vi "HFRR ADV v044.vi"() -> ()   [LabVIEW 2025] (continued)
          frame #3 {
          }
          frame #4 {
          }
          frame #5 {
          }
          frame #6 {
            # "CAL;END"
          }
          frame #7 {
            w857 = 0.0 ("x")
            w858 = 60.0 ("x")
            n824 = local read "Temperature diff"() -> (w861:dbl)
            n825 = local read "Air 60deg temp"() -> (w860:dbl)
            n826 = local read "Air 0deg temp"() -> (w859:dbl)
            n827 = Add(x=w858, y=w861) -> (x+y=w868:dbl)
            n828 = Subtract(x=w858, y=w861) -> (x-y=w867:dbl)
            n829 = Add(x=w857, y=w861) -> (x+y=w866:dbl)
            n830 = Subtract(x=w857, y=w861) -> (x-y=w865:dbl)
            n831 = In Range and Coerce(upper limit=w868, x=w860, lower limit=w867) -> (In Range?=w864:bool)  [unwired: 1 out]
            n832 = In Range and Coerce(upper limit=w866, x=w859, lower limit=w865) -> (In Range?=w863:bool)  [unwired: 1 out]
            n833 = And(x=w864, y=w863) -> (x .and. y?=w862:bool)
            n834 = case shown="True" w862 {
              frame False {
                n835 = property on="Accept & Save Air Temperature step 4" class="Bool (strict)"("DisabledEnum"=T19."Disabled" ("Disabled")) -> ()  [unwired: 2 in, 2 out]
                n836 = local write "Air Temperature Calibration"(enum32{"True", "Fail"}."Fail" ("Sample Temperature Calibration  2")) -> ()
              }
              frame True {
                n837 = local write "Air Temperature Calibration"(enum32{"True", "Fail"}."True" ("Sample Temperature Calibration  2")) -> ()
                n838 = property on="Accept & Save Air Temperature step 4" class="Bool (strict)"("DisabledEnum"=T19."Enabled" ("Disabled")) -> ()  [unwired: 2 in, 2 out]
              }
            }
          }
          frame #8 {
            # "CAL;END"
          }
          frame #9 {
            n839 = local write "Tab Control 4"(T14."Air Step 4" ("Tab Control 4")) -> ()
          }
        }
      }
      event "Back Stroke step main temperature": Value Change {
        n840 = event-data() -> ()  [unwired: 1 in, 6 out]
        n841 = stacked-sequence {
          frame #0 {
            n842 = Wait (ms)(milliseconds to wait=u32 1000) -> ()  [unwired: 1 out]
          }
          frame #1 {
            # "CAL;END"
            n843 = local write "Due Write"("CAL;END" ("Command")) -> ()
          }
          frame #2 {
            n844 = Wait (ms)(milliseconds to wait=u32 1000) -> ()  [unwired: 1 out]
          }
          frame #3 {
            # "CAL;END"
            n845 = local write "Due Write"("CAL;END" ("Command")) -> ()
          }
          frame #4 {
            n846 = local write "Temperature Selection"(T15."Default" ("Temperature Selection")) -> ()
            n847 = local write "Calibration Selection"(T10."Default" ("Calibration Selection")) -> ()
            n848 = local write "Main Calibration Tab"(T9."Main" ("Main Calibration Tab")) -> ()
            n849 = local write "Tab Control 4"(T14."Main" ("Tab Control 4")) -> ()
          }
        }
      }
      event "TEMPERATURE STEP  Back 4", "TEMPERATURE STEP 1 Back 3", "TEMPERATURE STEP  Back 3", "TEMPERATURE STEP 1 Back 2", "Back Air TEMPERATURE Step 4", "Back SAMPLE TEMPERATURE Step 4": Value Change {
        # "Back Stroke step main temperature"
        n850 = event-data() -> ()  [unwired: 1 in, 6 out]
        n851 = stacked-sequence {
          frame #0 {
            n852 = Wait (ms)(milliseconds to wait=u32 1000) -> ()  [unwired: 1 out]
          }
          frame #1 {
            # "CAL;END"
            n853 = local write "Due Write"("CAL;END" ("Command")) -> ()
          }
          frame #2 {
            n854 = Wait (ms)(milliseconds to wait=u32 1000) -> ()  [unwired: 1 out]
          }
          frame #3 {
            # "CAL;END"
            n855 = local write "Due Write"("CAL;END" ("Command")) -> ()
          }
          frame #4 {
            # "TEMPERATURE STEP  Back 4"
            n856 = local write "Main Calibration Tab"(T9."Temperature" ("Main Calibration Tab")) -> ()
            n857 = local write "Temperature Selection"(T15."Default" ("Temperature Selection")) -> ()
            n858 = local write "Tab Control 4"(T14."Main" ("Tab Control 4")) -> ()
            n859 = local write "Calibration Selection"(T10."Default" ("Calibration Selection")) -> ()
          }
        }
      }
      event "FF BACK", "FF BACK 2", "FF BACK 3", "FF BACK 4", "FF BACK 5", "FF BACK 6": Value Change {
        n860 = event-data() -> ()  [unwired: 1 in, 6 out]
        n861 = stacked-sequence {
          frame #0 {
            n862 = Wait (ms)(milliseconds to wait=u32 1000) -> ()  [unwired: 1 out]
          }
          frame #1 {
            n863 = local write "Due Write"("VC;0") -> ()
          }
          frame #2 {
            n864 = Wait (ms)(milliseconds to wait=u32 1000) -> ()  [unwired: 1 out]
          }
          frame #3 {
            n865 = local write "Due Write"("VC;0") -> ()
          }
          frame #4 {
            w894 = FALSE
            n866 = local write "FF BACK 2"(w894) -> ()
            n867 = local write "FF BACK 3"(w894) -> ()
            n868 = local write "FF BACK 4"(w894) -> ()
            n869 = local write "FF BACK 5"(w894) -> ()
            n870 = local write "FF BACK 6"(w894) -> ()
            n871 = local write "FF BACK"(w894) -> ()
          }
          frame #5 {
            n872 = local write "Temperature Selection"(T15."Default" ("Temperature Selection")) -> ()
            n873 = local write "Calibration Selection"(T10."Default" ("Calibration Selection")) -> ()
            n874 = local write "Friction Force Tab"(T13."Page 1" ("Friction Force Tab")) -> ()
            n875 = local write "Main Calibration Tab"(T9."Main" ("Main Calibration Tab")) -> ()
            n876 = property on="Tab Control 6" class="TabCtl (strict)"("Visible"=FALSE) -> ()  [unwired: 2 in, 2 out]
            n877 = property on="Friction Force Calibration Result Tab" class="TabCtl (strict)"("Visible"=FALSE) -> ()  [unwired: 2 in, 2 out]
          }
        }
      }
      event "Accept & Save FF": Value Change {
        n878 = event-data() -> ()  [unwired: 1 in, 6 out]
        n879 = stacked-sequence {
          frame #0 {
            n880 = Wait (ms)(milliseconds to wait=u32 1000) -> ()  [unwired: 1 out]
          }
          frame #1 {
            n881 = local write "Due Write"("VC;0") -> ()
          }
          frame #2 {
            n882 = Wait (ms)(milliseconds to wait=u32 1000) -> ()  [unwired: 1 out]
          }
          frame #3 {
            n883 = local write "Due Write"("VC;0") -> ()
          }
          frame #4 {
            w905 = FALSE
            n884 = local write "FF BACK 2"(w905) -> ()
            n885 = local write "FF BACK 3"(w905) -> ()
            n886 = local write "FF BACK 4"(w905) -> ()
            n887 = local write "FF BACK 5"(w905) -> ()
            n888 = local write "FF BACK 6"(w905) -> ()
            n889 = local write "FF BACK"(w905) -> ()
          }
          frame #5 {
            n890 = Get Date/Time In Seconds() -> (seconds since 1Jan1904=w908:timestamp)
            n891 = Format Into String(format string="%<%I:%M:%S:%p %d:%B:%Y>T", w908) -> (resulting string=w906:string)  [unwired: 2 in, 1 out]
            n892 = local write "FRICTION CALIBRATION"(w906) -> ()
          }
          frame #6 {
            n893 = local write "Temperature Selection"(T15."Default" ("Temperature Selection")) -> ()
            n894 = local write "Calibration Selection"(T10."Default" ("Calibration Selection")) -> ()
            n895 = local write "Friction Force Tab"(T13."Page 1" ("Friction Force Tab")) -> ()
            n896 = local write "Main Calibration Tab"(T9."Main" ("Main Calibration Tab")) -> ()
            n897 = local write "Save Button"(TRUE ("Save Button")) -> ()
            n898 = property on="Tab Control 6" class="TabCtl (strict)"("Visible"=FALSE) -> ()  [unwired: 2 in, 2 out]
            n899 = property on="Friction Force Calibration Result Tab" class="TabCtl (strict)"("Visible"=FALSE) -> ()  [unwired: 2 in, 2 out]
          }
        }
      }
      event "FF CONTINUE": Value Change {
        n900 = event-data() -> ()  [unwired: 1 in, 6 out]
        n901 = local write "FF CONTINUE"(FALSE ("FF CONTINUE")) -> ()
        n902 = local write "Friction Force Tab"(T13."Page 2" ("Friction Force Tab")) -> ()
      }
      event "FF CONTINUE 2": Value Change {
        n903 = event-data() -> ()  [unwired: 1 in, 6 out]
        n904 = local write "FF CONTINUE 2"(FALSE ("FF CONTINUE")) -> ()
        n905 = local write "Friction Force Tab"(T13."Page 3" ("Friction Force Tab")) -> ()
      }
      event "FF CONTINUE 3": Value Change {
        n906 = event-data() -> ()  [unwired: 1 in, 6 out]
        n907 = local write "FF CONTINUE 3"(FALSE ("FF CONTINUE")) -> ()
        n908 = local write "Friction Force Tab"(T13."Page 4" ("Friction Force Tab")) -> ()
      }
      event "FF CONTINUE 4": Value Change {
        n909 = event-data() -> ()  [unwired: 1 in, 6 out]
        n910 = local write "FF CONTINUE 4"(FALSE ("FF CONTINUE")) -> ()
        n911 = local write "Friction Force Tab"(T13."Page 5" ("Friction Force Tab")) -> ()
        n912 = property on="Friction Force Calibration Result Tab" class="TabCtl (strict)"("Visible"=FALSE) -> ()  [unwired: 2 in, 2 out]
      }
      event "FF CONTINUE 5": Value Change {
        n913 = event-data() -> ()  [unwired: 1 in, 6 out]
        n914 = local write "FF CONTINUE 5"(FALSE ("FF CONTINUE")) -> ()
        n915 = local write "Friction Force Tab"(T13."Page 6" ("Friction Force Tab")) -> ()
        n916 = property on="Friction Force Calibration Result Tab" class="TabCtl (strict)"("Visible"=FALSE) -> ()  [unwired: 2 in, 2 out]
        n917 = property on="Tab Control 6" class="TabCtl (strict)"("Visible"=FALSE) -> ()  [unwired: 2 in, 2 out]
      }
      event "Stroke Report Button": Value Change {
        n918 = event-data() -> ()  [unwired: 1 in, 6 out]
        n919 = local read "Point 5 - 1.0 mm"() -> (w930:bool)
        n920 = case shown="False" w930 {
          tunnel: [0.8 1.0] -> w929
          frame False {
          }
          frame True {
          }
        }
        n921 = local read "Machine Serial Number"() -> (w933:string)
        n922 = local read "USERNAME"() -> (w931:string)
        n923 = local write "Stroke Report Button"(FALSE ("Stroke Report Button")) -> ()
        n924 = call "Stroke Calibration Report.vi"("measured_value"=w929, "operator_name"=w931, "Instrument_serial Number"=w933) -> ()  [unwired: 7 in, 2 out]
      }
      event "Sample Report Button": Value Change {
        n925 = event-data() -> ()  [unwired: 1 in, 6 out]
        n926 = local read "Machine Serial Number"() -> (w939:string)
        n927 = local read "Sample 0deg temp"() -> (w936:dbl)
        n928 = local read "Sample 60deg temp"() -> (w937:dbl)
        n929 = local read "USERNAME"() -> (w938:string)
        n930 = call "Temperature Calibration Report.vi"("measured_60"=w937, "measured_zero"=w936, "operator_name"=w938, "Instrument_serial Number"=w939) -> ()  [unwired: 6 in, 2 out]
        n931 = local write "Sample Report Button"(FALSE ("Sample Report Button")) -> ()
      }
      event "Report Button FF": Value Change {
        n932 = event-data() -> ()  [unwired: 1 in, 6 out]
        n933 = local read "FF PASS"() -> (w944:bool)
        n934 = local read "Machine Serial Number"() -> (w947:string)
        n935 = Select(t="PASS", s=w944, f="FAIL") -> (s? t:f=w941:string)
        n936 = local read "USERNAME"() -> (w946:string)
        n937 = call "FF Calibration Report.vi"("pass_or_fail"=w941, "operator_name"=w946, "Instrument_serial Number"=w947) -> ()  [unwired: 7 in, 2 out]
        n938 = local write "Report Button FF"(FALSE ("Sample Report Button")) -> ()
      }
      event "Air Temperature Report Button": Value Change {
        n939 = event-data() -> ()  [unwired: 1 in, 6 out]
        n940 = local read "Machine Serial Number"() -> (w952:string)
        n941 = local read "Air 0deg temp"() -> (w949:dbl)
        n942 = local read "Air 60deg temp"() -> (w950:dbl)
        n943 = local read "USERNAME"() -> (w951:string)
        n944 = call "Air Temperature Calibration Report.vi"("measured_60"=w950, "measured_zero"=w949, "operator_name"=w951, "Instrument_serial Number"=w952) -> ()  [unwired: 6 in, 2 out]
        n945 = local write "Air Temperature Report Button"(FALSE ("Sample Report Button")) -> ()
      }
      event "Quit": Value Change {
        n946 = event-data() -> ()  [unwired: 1 in, 6 out]
      }
    }
    n947 = Wait (ms)(milliseconds to wait=u32 100) -> ()  [unwired: 1 out]
  }
  n948 = while {
    shift-right: [w955] -> _
    shift-left: "Enum - Selector" -> [w956]
    stop <- w957 stop-if-true
    # "Auto Start Logic Loop"
    n949 = case shown="\"Maintain Stage\"" w956 {
      tunnel: [w960 w966 w994 w1029 w1059 Auto_Start_enum."Exit" ("Enum - Selector") Auto_Start_enum."Init" ("Enum - Selector")] -> w955
      frame "Init", Default {
        n950 = local read "Auto Start Test"() -> (w959:bool)
        n951 = Select(t=Auto_Start_enum."Humidity & Temperature On" ("Enum - Selector"), s=w959, f=Auto_Start_enum."Init") -> (s? t:f=w960:T17)
      }
      frame "Humidity & Temperature On" {
        n952 = stacked-sequence {
          tunnel: [_ _ _ _ _ _ Auto_Start_enum."Reach point" ("Enum - Selector")] -> w963
          frame #0 {
            w968 = T19."Disabled and Grayed Out" ("Disabled")
            w969 = TRUE ("Heater Button")
            n953 = property on="Humidity" class="Bool (strict)"("DisabledEnum"=w968) -> ()  [unwired: 2 in, 2 out]
            n954 = property on="Heater Button" class="Bool (strict)"("DisabledEnum"=w968) -> ()  [unwired: 2 in, 2 out]
            n955 = local write "Heater Button"(w969) -> ()
            n956 = local write "Humidity"(w969) -> ()
            n957 = property on="Heater Button" class="Bool (strict)"("Val(Sgnl)"=TRUE ("Value (Signaling)")) -> ()  [unwired: 2 in, 2 out]
          }
          frame #1 {
            n958 = Wait (ms)(milliseconds to wait=u32 3000) -> ()  [unwired: 1 out]
          }
          frame #2 {
            n959 = local read "Set Temp"() -> (w975:dbl)
            n960 = Number To Fractional String(number=w975, precision (6)=i16 2) -> (F-format string=w972:string)  [unwired: 2 in]
            n961 = Concatenate Strings("ST;" ("Command"), w972) -> (w973:string)
            n962 = local write "Due Write"(w973) -> ()
          }
          frame #3 {
            n963 = Wait (ms)(milliseconds to wait=u32 1500) -> ()  [unwired: 1 out]
          }
          frame #4 {
            (unwired) i16 2 ("precision (6)")
            n964 = local read "WriteHumidity"() -> (w977:string[])
            n965 = local read "Set Rh"() -> (w980:dbl)
            n966 = Number To Fractional String(number=w980) -> (F-format string=w981:string)  [unwired: 3 in]
            n967 = Concatenate Strings("M;" ("new element/subarray"), w981) -> (w982:string)
            n968 = Insert Into Array(array=w977, new element=w982) -> (w978:string[])  [unwired: 1 in]
            n969 = local write "WriteHumidity"(w978) -> ()
            n970 = local write "Due Write"("HE;1" ("Command")) -> ()
          }
          frame #5 {
            n971 = Wait (ms)(milliseconds to wait=u32 1500) -> ()  [unwired: 1 out]
          }
          frame #6 {
            w985 = TRUE ("Reach point temp")
            n972 = local write "Reach point Humidity"(w985) -> ()
            n973 = local write "Reach point temp"(w985) -> ()
          }
        }
        n974 = local read "Auto Start Test"() -> (w965:bool)
        n975 = Not(x=w965) -> (.not. x?=w964:bool)
        n976 = Select(t=Auto_Start_enum."close", s=w964, f=w963) -> (s? t:f=w966:T17)
      }
      frame "Reach point" {
        w995 = TRUE ("PAUSE")
        w1003 = 1.0 ("y")
        w1006 = 1.0 ("y")
        n977 = local read "Set Temp"() -> (w988:dbl)
        n978 = local read "Set Humidity:"() -> (w1002:dbl)
        n979 = local read "Humidity ( %RH )"() -> (w1007:dbl)
        n980 = Add(x=w988, y=w1006) -> (x+y=w1005:dbl)
        n981 = Subtract(x=w988, y=w1006) -> (x-y=w1004:dbl)
        n982 = Add(x=w1002, y=w1003) -> (x+y=w1001:dbl)
        n983 = Subtract(x=w1002, y=w1003) -> (x-y=w1000:dbl)
        n984 = local read "TEMP"() -> (w1008:dbl)
        n985 = In Range and Coerce(upper limit=w1001, x=w1007, lower limit=w1000) -> (In Range?=w989:bool)  [unwired: 1 out]
        n986 = In Range and Coerce(upper limit=w1005, x=w1008, lower limit=w1004) -> (In Range?=w990:bool)  [unwired: 1 out]
        n987 = disable-structure shown="Enabled" {
          disable-tunnel: w989 -> [w1009 _]
          disable-tunnel: [w1009 TRUE] -> w987
          frame Disabled {
            n988 = case shown="True" w1009 {
              frame False {
              }
              frame True {
                n989 = case shown="True" "Reach point Humidity" {
                  selector: "Reach point Humidity" -> [_ w1015]
                  frame False {
                  }
                  frame True {
                    n990 = local read "EVENT LOG"() -> (w1012:string)
                    n991 = Not(x=w1015) -> (.not. x?=w1014:bool)
                    n992 = local write "Reach point Humidity"(w1014) -> ()
                    n993 = call "Event Log.vi"("Content"="Target Humidity reached", "EVENT LOG"=w1012) -> ("EVENT LOG"=w1013:string)  [unwired: 8 in, 1 out]
                    n994 = local write "EVENT LOG"(w1013) -> ()
                  }
                }
              }
            }
          }
          frame Enabled {
          }
        }
        n995 = case shown="True" w990 {
          frame False {
          }
          frame True {
            n996 = case shown="True" "Reach point temp" {
              selector: "Reach point temp" -> [_ w1022]
              frame False {
              }
              frame True {
                n997 = local read "EVENT LOG"() -> (w1019:string)
                n998 = Not(x=w1022) -> (.not. x?=w1021:bool)
                n999 = local write "Reach point temp"(w1021) -> ()
                n1000 = call "Event Log.vi"("Content"="Target Temperature reached", "EVENT LOG"=w1019) -> ("EVENT LOG"=w1020:string)  [unwired: 8 in, 1 out]
                n1001 = local write "EVENT LOG"(w1020) -> ()
              }
            }
          }
        }
        n1002 = local read "Auto Start Test"() -> (w993:bool)
        n1003 = And(x=w990, y=w987) -> (x .and. y?=w999:bool)
        n1004 = Select(t=Auto_Start_enum."Maintain Stage" ("Enum - Selector"), s=w999, f=Auto_Start_enum."Reach point" ("Enum - Selector")) -> (s? t:f=w996:T17)
        n1005 = Not(x=w993) -> (.not. x?=w992:bool)
        n1006 = Select(t=Auto_Start_enum."close", s=w992, f=w996) -> (s? t:f=w994:T17)
        n1007 = call "ELAPSED TIMER VI.vi"("RESET"=w995, "PAUSE"=w995) -> ()  [unwired: 7 in, 3 out]
      }
      frame "Maintain Stage" {
        w1037 = 2.0 ("y")
        w1036 = 1.0 ("y")
        # "Humidity and temperature set point has stabilized."
        # "Humidity and  temperatures Set Point  have been reached"
        n1008 = local read "Set Temp"() -> (w1024:dbl)
        n1009 = local read "Set Humidity:"() -> (w1040:dbl)
        n1010 = local read "Humidity ( %RH )"() -> (w1043:dbl)
        n1011 = Add(x=w1024, y=w1036) -> (x+y=w1042:dbl)
        n1012 = Subtract(x=w1024, y=w1036) -> (x-y=w1041:dbl)
        n1013 = local read "TEMP"() -> (w1044:dbl)
        n1014 = Add(x=w1040, y=w1037) -> (x+y=w1039:dbl)
        n1015 = Subtract(x=w1040, y=w1037) -> (x-y=w1038:dbl)
        n1016 = In Range and Coerce(upper limit=w1042, x=w1044, lower limit=w1041) -> (In Range?=w1035:bool)  [unwired: 1 out]
        n1017 = In Range and Coerce(upper limit=w1039, x=w1043, lower limit=w1038) -> ()  [unwired: 2 out]
        n1018 = And(x=w1035, y=TRUE) -> (x .and. y?=w1034:bool)
        n1019 = Not(x=w1034) -> (.not. x?=w1033:bool)
        n1020 = call "ELAPSED TIMER VI.vi"("TARGET"=60.0, "RESET"=w1033, "PAUSE"=FALSE) -> ("ELAPSED INDICATION"=w1030:bool)  [unwired: 6 in, 2 out]
        n1021 = case shown="True" w1030 {
          tunnel: w1030 -> [_ w1047]
          tunnel: [Auto_Start_enum."Maintain Stage" ("Enum - Selector") w1046] -> w1028
          frame False {
          }
          frame True {
            n1022 = stacked-sequence {
              tunnel: w1047 -> [_ _ _ _ _]
              tunnel: [_ _ _ _ Auto_Start_enum."Start Stage" ("Enum - Selector")] -> w1046
              frame #0 {
                n1023 = local read "EVENT LOG"() -> (w1049:string)
                n1024 = call "Event Log.vi"("Content"="Temperature set point has stabilized.", "EVENT LOG"=w1049) -> ("EVENT LOG"=w1050:string)  [unwired: 8 in, 1 out]
                n1025 = local write "EVENT LOG"(w1050) -> ()
              }
              frame #1 {
                n1026 = Wait (ms)(milliseconds to wait=u32 100) -> ()  [unwired: 1 out]
              }
              frame #2 {
                n1027 = local read "EVENT LOG"() -> (w1054:string)
                n1028 = call "Event Log.vi"("Content"="Auto Test Started", "EVENT LOG"=w1054) -> ("EVENT LOG"=w1055:string)  [unwired: 8 in, 1 out]
                n1029 = local write "EVENT LOG"(w1055) -> ()
                n1030 = local write "FRICVALZ 4"(TRUE ("FRICVALZ 4")) -> ()
              }
              frame #3 {
                w1056 = TRUE ("RUN")
                n1031 = local write "RUN"(w1056) -> ()
                n1032 = property on="Auto Start Temp" class="Bool (strict)"("Val(Sgnl)"=w1056) -> ()  [unwired: 2 in, 2 out]
                "Auto Start Temp" <- w1056
              }
              frame #4 {
              }
            }
          }
        }
        n1033 = local read "Auto Start Test"() -> (w1027:bool)
        n1034 = Not(x=w1027) -> (.not. x?=w1026:bool)
        n1035 = Select(t=Auto_Start_enum."close", s=w1026, f=w1028) -> (s? t:f=w1029:T17)
      }
      frame "Start Stage" {
        w1058 = TRUE ("PAUSE")
        n1036 = local read "Auto Start Test"() -> (w1063:bool)
        n1037 = Not(x=w1063) -> (.not. x?=w1062:bool)
        n1038 = Select(t=Auto_Start_enum."close" ("Enum - Selector"), s=w1062, f=Auto_Start_enum."Start Stage" ("Enum - Selector")) -> (s? t:f=w1059:T17)
        n1039 = call "ELAPSED TIMER VI.vi"("RESET"=w1058, "PAUSE"=w1058) -> ()  [unwired: 7 in, 3 out]
      }
      frame "close" {
        w1066 = FALSE ("Heater Button")
        n1040 = local write "RUN"(w1066) -> ()
        n1041 = local write "Heater Button"(w1066) -> ()
        n1042 = local write "Humidity"(w1066) -> ()
        n1043 = local write "Auto Start Test"(w1066) -> ()
        n1044 = property on="Heater Button" class="Bool (strict)"("Val(Sgnl)"=FALSE ("Value (Signaling)")) -> ()  [unwired: 2 in, 2 out]
        n1045 = local write "Humidity 2"(TRUE ("Humidity")) -> ()
      }
      frame "Exit" {
      }
    }
    n1046 = Wait (ms)(milliseconds to wait=u32 100) -> ()  [unwired: 1 out]
    n1047 = local read "Quit"() -> (w957:bool)
  }
  n1048 = property on="Service Password Log" class="Str"("Visible"=w26) -> ()  [unwired: 2 in, 2 out]
  n1049 = property on="Password 3" class="Clust (strict)"("Visible"=w26) -> ()  [unwired: 2 in, 2 out]
  n1050 = while {
    stop <- w1095 stop-if-true
    w1078 = errorcluster {"status"=FALSE, "code"=0, "source"=""} ("error in (no error) 3")
    # "this loop is for manual report generation"
    n1051 = local read "Confirm Measrurement"() -> (w1077:bool)
    n1052 = case shown="True" w1077 {
      selector: w1077 -> [_ w1185]
      tunnel: errorcluster {"status"=FALSE, "code"=0, "source"=""} ("error in (no error) 3") -> [_ w1186]
      tunnel: [_ w1184] -> _
      frame False {
      }
      frame True {
        n1053 = stacked-sequence {
          tunnel: w1186 -> [_ w1219 _]
          tunnel: w1185 -> [_ _ w1326]
          tunnel: [_ w1207 _] -> w1184
          frame #0 {
            n1054 = String To Path(string="C:\\LAB-IQ\\Image Calibrate v01.dcf") -> (path=w1189:path)
            n1055 = Open/Create/Replace File ("Open File")(file path (use dialog)=w1189) -> (refnum out=w1190:refnum<file>)  [unwired: 5 in, 2 out]
            n1056 = for {
              N: 4 -> [_]
              tunnel: w1190 -> [w1196]
              i -> [w1192]
              n1057 = Read from Text File ("Read File")(file (use dialog)=w1196) -> (text=w1197:string)  [unwired: 3 in, 3 out]
              n1058 = String Subset(string=w1197, offset (0)=6, length (rest)=10 ("length (rest)")) -> (substring=w1193:string)
              n1059 = Fract/Exp String To Number(string=w1193) -> (number=w1191:dbl)  [unwired: 3 in, 1 out]
              n1060 = case shown="3" w1192 {
                tunnel: w1191 -> [w1198 w1199 _ w1200 _]
                frame 0 {
                  n1061 = local write "5x Gain"(w1198) -> ()
                }
                frame 1 {
                  n1062 = local write "10x Gain"(w1199) -> ()
                }
                frame 2 {
                }
                frame 3 {
                  n1063 = local write "100x gain"(w1200) -> ()
                }
                frame 4, Default {
                }
              }
            }
          }
          frame #1 {
            n1064 = local read "TEST STANDARD"() -> (w1202:T5)
            n1065 = case shown="\"ISO 12156\"" w1202 {
              tunnel: ["ASTM D6079" "ISO 12156"] -> w1201
              frame "ASTM D6079", Default {
              }
              frame "ISO 12156" {
              }
            }
            n1066 = call "IMAGE ANALYSIS.vi"("Enum"=POST_ANALYSIS_ENUM."GET MEASUREMENTS", "error in"=w1219) -> ("error out"=w1226:errorcluster)  [unwired: 8 in, 1 out]
            n1067 = local read "Magnification :"() -> (w1212:string)
            n1068 = call "Stall Data Flow.vim"("value in"=w1226, "milliseconds to wait"=u32 1000) -> ("value out"=w1225:errorcluster)  [unwired: 1 out]
            n1069 = local read "Test File List :"() -> (w1223:string)
            n1070 = case shown="\"10x\"" w1212 {
              tunnel: [w1262 w1263] -> w1210
              frame "5x", Default {
                n1071 = local read "5x Gain"() -> (w1262:dbl)
              }
              frame "10x" {
                # "5x"
                n1072 = local read "10x Gain"() -> (w1263:dbl)
              }
            }
            n1073 = call "IMAGE ANALYSIS.vi"("Enum"=POST_ANALYSIS_ENUM."READ", "error in"=w1225) -> ("error out"=w1222:errorcluster, "data out"=w1213:string)  [unwired: 8 in]
            n1074 = Match Pattern(string=w1213, regular expression="\"type\": ") -> (after substring=w1217:string)  [unwired: 1 in, 3 out]
            n1075 = call "IMAGE PATH CREATION PY.vi"("error in (no error)"=w1222, "File Name :"=w1223) -> ("error out"=w1221:errorcluster, "File Path"=w1209:path, "File Path String:"=w1204:string)  [unwired: 7 in]
            n1076 = Match Pattern(string=w1217, regular expression=",") -> (before substring=w1203:string)  [unwired: 1 in, 3 out]
            n1077 = local read "Calibration Tab"() -> (w1206:enum32{"Measrument", "Calibrate"})
            n1078 = call "Stall Data Flow.vim"("value in"=w1221, "milliseconds to wait"=u32 250) -> ("value out"=w1205:errorcluster)  [unwired: 1 out]
            n1079 = Equal?(x=w1203, y="\"rectangle\"") -> (x = y?=w1214:bool)
            n1080 = case shown="False" w1214 {
              tunnel: w1213 -> [w1268 w1323]
              tunnel: w1210 -> [_ w1314]
              tunnel: cluster{"major":dbl, "minor":dbl, "average":dbl} {"major"=0.0, "minor"=0.0, "average"=0.0} -> [w1266 w1310]
              tunnel: [w1265 w1307] -> w1208
              tunnel: w1203 -> [w1267 _]
              tunnel: w1210 -> [w1264 _]
              frame False {
                n1081 = Equal?(x=w1267, y="\"line\"") -> (x = y?=w1269:bool)
                n1082 = case shown="True" w1269 {
                  tunnel: w1268 -> [_ w1284]
                  tunnel: w1266 -> [w1271 w1283]
                  tunnel: [w1271 w1281] -> w1265
                  tunnel: w1264 -> [_ w1280]
                  frame False {
                  }
                  frame True {
                    w1279 = 0.0 ("Major Axis")
                    n1083 = Match Pattern(string=w1284, regular expression="\"length_px\":") -> (after substring=w1282:string)  [unwired: 1 in, 3 out]
                    n1084 = property on="Major Axis" class="DigNum (strict)"("Caption.Text"="") -> ()  [unwired: 2 in, 2 out]
                    n1085 = property on="Minor Axis" class="DigNum (strict)"("Caption.Text"="") -> ()  [unwired: 2 in, 2 out]
                    n1086 = property on="Average" class="DigNum (strict)"("Caption.Text"="Line") -> ()  [unwired: 2 in, 2 out]
                    n1087 = Fract/Exp String To Number(string=w1282, default (0 dbl)=0.0 ("default (0 DBL)")) -> (number=w1278:dbl)  [unwired: 2 in, 1 out]
                    "Pixel Value" <- w1278
                    n1088 = Multiply(x=w1278, y=w1280) -> (x*y=w1291:dbl)
                    n1089 = Multiply(x=w1291, y=1000.0) -> (x*y=w1274:dbl)
                    n1090 = Divide(x=w1274, y=1000.0) -> (x/y=w1277:dbl)
                    n1091 = local write "Measurment (mm)"(w1277) -> ()
                    n1092 = Bundle By Name(cluster=w1283, "average"=w1274) -> (w1281:cluster{"major":dbl, "minor":dbl, "average":dbl})
                    n1093 = Number To Fractional String(number=w1274, precision (6)=i16 1) -> (F-format string=w1273:string)  [unwired: 2 in]
                    n1094 = local write "Minor Axis"(w1279) -> ()
                    n1095 = local write "Major Axis"(w1279) -> ()
                    n1096 = Fract/Exp String To Number(string=w1273) -> (number=w1272:dbl)  [unwired: 3 in, 1 out]
                    n1097 = local write "Average"(w1272) -> ()
                  }
                }
              }
              frame True {
                w1311 = 1000.0 ("y")
                w1317 = 0.0 ("default (0 DBL)")
                n1098 = Match Pattern(string=w1323, regular expression=" \"width_px\":") -> (after substring=w1321:string)  [unwired: 1 in, 3 out]
                n1099 = Match Pattern(string=w1321, regular expression="\"height_px\":") -> (before substring=w1319:string, after substring=w1318:string)  [unwired: 1 in, 2 out]
                n1100 = Fract/Exp String To Number(string=w1319, default (0 dbl)=w1317) -> (number=w1316:dbl)  [unwired: 2 in, 1 out]
                n1101 = Fract/Exp String To Number(string=w1318, default (0 dbl)=w1317) -> (number=w1315:dbl)  [unwired: 2 in, 1 out]
                n1102 = Multiply(x=w1316, y=w1314) -> (x*y=w1313:dbl)
                n1103 = Multiply(x=w1315, y=w1314) -> (x*y=w1312:dbl)
                n1104 = Multiply(x=w1313, y=w1311) -> (x*y=w1297:dbl)
                n1105 = Multiply(x=w1312, y=w1311) -> (x*y=w1295:dbl)
                n1106 = Add(x=w1297, y=w1295) -> (x+y=w1309:dbl)
                n1107 = property on="Major Axis" class="DigNum (strict)"("Caption.Text"="Major Axis") -> ()  [unwired: 2 in, 2 out]
                n1108 = property on="Minor Axis" class="DigNum (strict)"("Caption.Text"="Minor Axis") -> ()  [unwired: 2 in, 2 out]
                n1109 = property on="Average" class="DigNum (strict)"("Caption.Text"="Average") -> ()  [unwired: 2 in, 2 out]
                n1110 = Divide(x=w1309, y=2.0) -> (x/y=w1293:dbl)
                n1111 = Bundle By Name(cluster=w1310, "major"=w1297, "minor"=w1295, "average"=w1293) -> (w1307:cluster{"major":dbl, "minor":dbl, "average":dbl})
                n1112 = Number To Fractional String(number=w1295, precision (6)=i16 1) -> (F-format string=w1302:string)  [unwired: 2 in]
                n1113 = Number To Fractional String(number=w1293, precision (6)=i16 1) -> (F-format string=w1303:string)  [unwired: 2 in]
                n1114 = Number To Fractional String(number=w1297, precision (6)=i16 1) -> (F-format string=w1301:string)  [unwired: 2 in]
                n1115 = Fract/Exp String To Number(string=w1302) -> (number=w1294:dbl)  [unwired: 3 in, 1 out]
                n1116 = Fract/Exp String To Number(string=w1303) -> (number=w1292:dbl)  [unwired: 3 in, 1 out]
                n1117 = Fract/Exp String To Number(string=w1301) -> (number=w1296:dbl)  [unwired: 3 in, 1 out]
                n1118 = local write "Major Axis"(w1296) -> ()
                n1119 = local write "Average"(w1292) -> ()
                n1120 = local write "Minor Axis"(w1294) -> ()
              }
            }
            n1121 = case shown="\"Measrument\", Default" w1206 {
              tunnel: w1209 -> [w1236 _]
              tunnel: w1208 -> [w1235 _]
              tunnel: [w1232 w1261] -> w1207
              tunnel: w1205 -> [w1234 w1261]
              tunnel: w1204 -> [w1233 _]
              tunnel: w1201 -> [w1231 _]
              frame "Measrument", Default {
                n1122 = stacked-sequence {
                  tunnel: w1236 -> [w1254 _]
                  tunnel: w1235 -> [w1252 _]
                  tunnel: w1234 -> [w1250 _]
                  tunnel: w1233 -> [w1249 _]
                  tunnel: [w1244 _] -> w1232
                  tunnel: w1231 -> [w1237 _]
                  frame #0 {
                    n1123 = call "IMAGE ANALYSIS.vi"("Enum"=POST_ANALYSIS_ENUM."SAVE IMAGE", "error in"=w1250, "IMAGE FILE PATH"=w1249) -> ("error out"=w1248:errorcluster)  [unwired: 7 in, 1 out]
                    n1124 = call "Stall Data Flow.vim"("value in"=w1248, "milliseconds to wait"=u32 1000) -> ("value out"=w1239:errorcluster)  [unwired: 1 out]
                    n1125 = local read "Test File List :"() -> (w1256:string)
                    n1126 = call "IMAGE ANALYSIS.vi"("Enum"=POST_ANALYSIS_ENUM."MINIMIZE UI", "error in"=w1239) -> ("error out"=w1246:errorcluster)  [unwired: 8 in, 1 out]
                    n1127 = Bundle By Name(cluster=T26 {"File Name"="", "Test Method"="", "Operator"="", "Fuel Description"="", "Date and time"=""} ("Main Ref"), "Test Method"=w1237, "File Name"=w1256) -> (w1257:T26)
                    n1128 = call "Stall Data Flow.vim"("value in"=w1246, "milliseconds to wait"=u32 1500) -> ("value out"=w1241:errorcluster)  [unwired: 1 out]
                    n1129 = call "duf file read.vi"("error in (no error)"=w1241, "Main Ref"=w1257) -> ("error out"=w1255:errorcluster, "Main Ref 2"=w1253:T26)  [unwired: 8 in]
                    n1130 = call "DETECTION REPORT for manual.vi"("error in (no error)"=w1255, "return value 3"=w1252, "Image File Path"=w1254, "Main Ref"=w1253) -> ("error out"=w1251:errorcluster)  [unwired: 7 in]
                    n1131 = call <vilib>:"Clear Errors.vi"("error in (no error)"=w1251) -> ("error out"=w1242:errorcluster)  [unwired: 5 in, 1 out]
                    n1132 = call "IMAGE ANALYSIS.vi"("Enum"=POST_ANALYSIS_ENUM."MINIMIZE UI", "error in"=w1242) -> ("error out"=w1244:errorcluster)  [unwired: 8 in, 1 out]
                  }
                  frame #1 {
                    n1133 = local write "Main Tab"(T4."HOME" ("Main Tab")) -> ()
                    n1134 = local write "Main Dashboard Buttons"(T1."Home" ("Main Dashboard Buttons")) -> ()
                  }
                }
              }
              frame "Calibrate" {
              }
            }
          }
          frame #2 {
            n1135 = Not(x=w1326) -> (.not. x?=w1325:bool)
            n1136 = local write "Confirm Measrurement"(w1325) -> ()
            n1137 = local read "Calibration Tab"() -> (w1324:enum32{"Measrument", "Calibrate"})
            n1138 = case shown="\"Measrument\", Default" w1324 {
              frame "Measrument", Default {
                (unwired) T21."HOME" ("Main Tab")
                n1139 = local write "Main Tab"(T4."HOME" ("Main Tab")) -> ()
              }
              frame "Calibrate" {
              }
            }
          }
        }
      }
    }
    n1140 = local read "Humidity"() -> (w1069:bool)
    n1141 = local read "Save Change"() -> (w1074:bool)
    n1142 = local read "Calibrate"() -> (w1075:bool)
    n1143 = local read "Auto Start Test"() -> (w1070:bool)
    n1144 = case shown="True" w1075 {
      selector: w1075 -> [_ w1182]
      frame False {
      }
      frame True {
        n1145 = Not(x=w1182) -> (.not. x?=w1181:bool)
        n1146 = local write "Calibrate"(w1181) -> ()
        n1147 = local write "Calibration Tab"(enum32{"Measrument", "Calibrate"}."Calibrate" ("Calibration Tab")) -> ()
      }
    }
    n1148 = case shown="True" w1074 {
      selector: w1074 -> [_ w1126]
      frame False {
      }
      frame True {
        n1149 = stacked-sequence {
          tunnel: w1126 -> [_ _ _ _ w1180]
          frame #0 {
            n1150 = call "IMAGE ANALYSIS.vi"("Enum"=POST_ANALYSIS_ENUM."HIDE UI") -> ()  [unwired: 9 in, 2 out]
          }
          frame #1 {
            n1151 = local read "100x gain"() -> (w1128:dbl)
            n1152 = local read "10x Gain"() -> (w1129:dbl)
            n1153 = local read "5x Gain"() -> (w1130:dbl)
            n1154 = Number To Fractional String(number=w1129, width (-)=i16 4, precision (6)=i16 7) -> (F-format string=w1151:string)  [unwired: 1 in]
            n1155 = Number To Fractional String(number=0.0, width (-)=i16 4, precision (6)=i16 7) -> (F-format string=w1146:string)  [unwired: 1 in]
            n1156 = Number To Fractional String(number=w1128, width (-)=i16 4, precision (6)=i16 7) -> (F-format string=w1134:string)  [unwired: 1 in]
            n1157 = Number To Fractional String(number=w1130, width (-)=i16 10 ("precision (6)"), precision (6)=i16 7) -> (F-format string=w1160:string)  [unwired: 1 in]
            n1158 = Concatenate Strings("[CH1]" ("string"), w1160, " - 5x Gain" ("string"), "\r") -> (w1150:string)
            n1159 = Concatenate Strings("[CH2]" ("string"), w1151, " - 10x Gain" ("string"), "\r") -> (w1149:string)
            n1160 = Concatenate Strings("[CH3]" ("string"), w1146, " - 20x Gain" ("string"), "\r") -> (w1140:string)
            n1161 = Concatenate Strings("[CH4]" ("string"), w1134, " - 100x Gain" ("string"), "\r") -> (w1133:string)
            n1162 = String To Path(string="C:\\LAB-IQ\\Image Calibrate v01.dcf") -> (path=w1163:path)
            n1163 = Concatenate Strings(w1150, w1149, w1140, w1133) -> (w1148:string)
            n1164 = call <vilib>:"Write Characters To File.vi"("append to file? (new file:F)"=FALSE, "character string"=w1148, "file path (dialog if empty)"=w1163) -> ()  [unwired: 2 in, 1 out]
          }
          frame #2 {
            n1165 = String To Path(string="C:\\LAB-IQ\\Image Calibrate v01.dcf") -> (path=w1166:path)
            n1166 = Open/Create/Replace File ("Open File")(file path (use dialog)=w1166) -> (refnum out=w1167:refnum<file>)  [unwired: 5 in, 2 out]
            n1167 = for {
              N: 4 -> [_]
              tunnel: w1167 -> [w1173]
              i -> [w1169]
              n1168 = Read from Text File ("Read File")(file (use dialog)=w1173) -> (text=w1174:string)  [unwired: 3 in, 3 out]
              n1169 = String Subset(string=w1174, offset (0)=6, length (rest)=10 ("length (rest)")) -> (substring=w1170:string)
              n1170 = Fract/Exp String To Number(string=w1170) -> (number=w1168:dbl)  [unwired: 3 in, 1 out]
              n1171 = case shown="3" w1169 {
                tunnel: w1168 -> [w1175 w1176 _ w1177 _]
                frame 0 {
                  n1172 = local write "5x Gain"(w1175) -> ()
                }
                frame 1 {
                  n1173 = local write "10x Gain"(w1176) -> ()
                }
                frame 2 {
                }
                frame 3 {
                  n1174 = local write "100x gain"(w1177) -> ()
                }
                frame 4, Default {
                }
              }
            }
          }
          frame #3 {
            n1175 = call "IMAGE ANALYSIS.vi"("Enum"=POST_ANALYSIS_ENUM."SHOW UI") -> ()  [unwired: 9 in, 2 out]
          }
          frame #4 {
            n1176 = Not(x=w1180) -> (.not. x?=w1179:bool)
            n1177 = local write "Save Change"(w1179) -> ()
          }
        }
      }
    }
    n1178 = case shown="False" w1070 {
      tunnel: w1069 -> [w1096 _]
      frame False {
        n1179 = case shown="True" w1096 {
          frame False {
          }
          frame True {
            n1180 = local read "Set Humidity:"() -> (w1100:dbl)
            n1181 = local read "Set Humidity:"() -> (w1103:dbl)
            n1182 = local read "Humidity ( %RH )"() -> (w1104:dbl)
            n1183 = Subtract(x=w1100, y=2.0) -> (x-y=w1098:dbl)
            n1184 = Add(x=w1103, y=2.0) -> (x+y=w1099:dbl)
            n1185 = In Range and Coerce(upper limit=w1099, x=w1104, lower limit=w1098) -> (In Range?=w1097:bool)  [unwired: 1 out]
            n1186 = case shown="True" w1097 {
              frame False {
              }
              frame True {
                n1187 = case shown="True" "Manual Humididty Reached" {
                  selector: "Manual Humididty Reached" -> [_ w1107]
                  frame False {
                  }
                  frame True {
                    n1188 = Not(x=w1107) -> (.not. x?=w1106:bool)
                    n1189 = local write "Manual Humididty Reached"(w1106) -> ()
                    n1190 = local read "EVENT LOG"() -> (w1109:string)
                    n1191 = call "Event Log.vi"("Content"="Target Humidity reached", "EVENT LOG"=w1109) -> ("EVENT LOG"=w1108:string)  [unwired: 8 in, 1 out]
                    n1192 = local write "EVENT LOG"(w1108) -> ()
                  }
                }
              }
            }
          }
        }
      }
      frame True {
        n1193 = local write "Manual Humididty Reached"(TRUE ("Manual Humididty Reached")) -> ()
      }
    }
    n1194 = local read "Cap Live Image"() -> (w1090:bool)
    n1195 = local read "SCAR MEASURMENT"() -> (w1093:enum32{"Auto Scar", "Manual Scar"})
    n1196 = Equal?(x=w1093, y=enum32{"Auto Scar", "Manual Scar"}."Manual Scar" ("SCAR MEASURMENT")) -> (x = y?=w1091:bool)
    n1197 = And(x=w1091, y=w1090) -> (x .and. y?=w1089:bool)
    n1198 = Wait (ms)(milliseconds to wait=u32 250) -> ()  [unwired: 1 out]
    n1199 = case shown="True" w1089 {
      selector: w1089 -> [_ w1412]
      frame False {
      }
      frame True {
        n1200 = stacked-sequence {
          tunnel: [_ _ _ w1431 _] -> _
          tunnel: w1412 -> [_ _ _ _ w1438]
          frame #0 {
            w1413 = 0.0
            n1201 = local write "Major Axis"(w1413) -> ()
            n1202 = local write "Minor Axis"(w1413) -> ()
            n1203 = local write "Average"(w1413) -> ()
          }
          frame #1 {
            n1204 = call "CAMERA LIVE FEED FGV.vi"("Enum - Menu"=CAMERA_LIVE_FEED_ENUM."CAMERA MINIMIZE") -> ()  [unwired: 9 in, 2 out]
          }
          frame #2 {
            n1205 = local read "Magnification len live scar"() -> (w1417:string)
            n1206 = case shown="\"10x\", Default" w1417 {
              tunnel: ["_10x" "_5x"] -> w1416
              frame "10x", Default {
              }
              frame "5x" {
              }
            }
            n1207 = local read "FILE 3"() -> (w1423:string)
            n1208 = call <vilib>:"Trim Whitespace.vi"("string"="C:\\LAB-IQ\\images\\") -> ("trimmed string"=w1425:string)  [unwired: 1 in]
            n1209 = String To Path(string=w1425) -> (path=w1424:path)
            n1210 = Concatenate Strings(w1423, w1416, ".png" ("string")) -> (w1422:string)
            n1211 = Build Path(base path=w1424, name or relative path=w1422) -> (appended path=w1421:path)
            n1212 = Path To String(path=w1421) -> (string=w1420:string)
            n1213 = call "CAMERA LIVE FEED FGV.vi"("Enum - Menu"=CAMERA_LIVE_FEED_ENUM."CAMERA SAVE", "Image Path"=w1420) -> ("error out"=w1418:errorcluster)  [unwired: 8 in, 1 out]
            n1214 = case shown="No Error" w1418 {
              frame No Error {
                n1215 = One Button Dialog(message="Image saved successfully") -> ()  [unwired: 1 in, 1 out]
              }
              frame Error {
              }
            }
          }
          frame #3 {
            n1216 = call "LIST FILE NAMES.vi"() -> ("error out"=w1433:errorcluster, "filenames"=w1430:string[])  [unwired: 10 in]
            n1217 = call "IMAGE ANALYSIS.vi"("Enum"=POST_ANALYSIS_ENUM."SHOW UI", "error in"=w1433) -> ("error out"=w1431:errorcluster)  [unwired: 8 in, 1 out]
            n1218 = property on="Test File List :" class="CmbBox"("Strings[]"=w1430) -> ()  [unwired: 2 in, 2 out]
          }
          frame #4 {
            (unwired) T25."Report" ("Main Dashboard Buttons")
            (unwired) T27."Report" ("Main Dashboard Buttons")
            n1219 = Not(x=w1438) -> (.not. x?=w1437:bool)
            n1220 = local write "Zoom Factore"(0.0 ("Zoom Factore")) -> ()
            n1221 = local write "Cap Live Image"(w1437) -> ()
            n1222 = local write "Main Tab"(T4."Adv Scar Report" ("Main Tab")) -> ()
            n1223 = property on="Cap Live Image" class="Bool (strict)"("BoolText.Text"="Capture Image" ("Boolean Text.Text")) -> ()  [unwired: 2 in, 2 out]
            n1224 = local write "Main Dashboard Buttons"(T1."Report" ("Main Dashboard Buttons")) -> ()
          }
        }
      }
    }
    n1225 = local read "change Gain"() -> (w1073:bool)
    n1226 = local read "Back Square"() -> (w1072:bool)
    n1227 = case shown="True" w1073 {
      selector: w1073 -> [_ w1117]
      frame False {
      }
      frame True {
        n1228 = stacked-sequence {
          tunnel: w1117 -> [_ w1125]
          frame #0 {
            n1229 = local read "Actual (µm)"() -> (w1121:dbl)
            n1230 = local read "Pixel Value"() -> (w1120:dbl)
            n1231 = local read "Magnification :"() -> (w1119:string)
            n1232 = Divide(x=w1121, y=w1120) -> (x/y=w1118:dbl)
            n1233 = case shown="\"10x\"" w1119 {
              tunnel: w1118 -> [w1122 w1123]
              frame "10x" {
                n1234 = local write "10x Gain"(w1122) -> ()
              }
              frame "5x", Default {
                n1235 = local write "5x Gain"(w1123) -> ()
              }
            }
          }
          frame #1 {
            n1236 = Not(x=w1125) -> (.not. x?=w1124:bool)
            n1237 = local write "change Gain"(w1124) -> ()
          }
        }
      }
    }
    n1238 = case shown="True" w1072 {
      selector: w1072 -> [_ w1115]
      frame False {
      }
      frame True {
        n1239 = Not(x=w1115) -> (.not. x?=w1114:bool)
        n1240 = local write "Back Square"(w1114) -> ()
        n1241 = local write "Calibration Tab"(enum32{"Measrument", "Calibrate"}."Measrument" ("Calibration Tab")) -> ()
      }
    }
    n1242 = local read "Rectangle Tool"() -> (w1084:bool)
    n1243 = local read "Clear ROI Tool"() -> (w1083:bool)
    n1244 = local read "Open Image"() -> (w1088:bool)
    n1245 = local read "line tool"() -> (w1085:bool)
    n1246 = local read "OUT"() -> (w1086:bool)
    n1247 = local read "In"() -> (w1087:bool)
    n1248 = case shown="True" w1088 {
      selector: w1088 -> [_ w1398]
      tunnel: [w1389 w1400] -> _
      tunnel: w1078 -> [w1389 w1399]
      frame False {
      }
      frame True {
        w1393 = "_5x" ("regular expression")
        n1249 = Not(x=w1398) -> (.not. x?=w1397:bool)
        n1250 = local write "Open Image"(w1397) -> ()
        n1251 = call "IMAGE ANALYSIS.vi"("Enum"=POST_ANALYSIS_ENUM."HIDE UI", "error in"=w1399) -> ("error out"=w1407:errorcluster)  [unwired: 8 in, 1 out]
        n1252 = call <vilib>:"Clear Errors.vi"("error in (no error)"=w1407) -> ("error out"=w1390:errorcluster)  [unwired: 5 in, 1 out]
        n1253 = call "File Dialog"("start path"=path "C:/LAB-IQ/images", "error in"=w1390) -> ("selected path"=w1392:path, "error out"=w1405:errorcluster)  [unwired: 10 in, 2 out]
        "Image path  2" <- w1392
        n1254 = call <vilib>:"Clear Errors.vi"("error in (no error)"=w1405) -> ("error out"=w1404:errorcluster)  [unwired: 5 in, 1 out]
        n1255 = call "IMAGE ANALYSIS.vi"("Enum"=POST_ANALYSIS_ENUM."OPEN FILE", "error in"=w1404, "File Path"=w1392) -> ("error out"=w1403:errorcluster)  [unwired: 7 in, 1 out]
        n1256 = call <vilib>:"Clear Errors.vi"("error in (no error)"=w1403) -> ("error out"=w1402:errorcluster)  [unwired: 5 in, 1 out]
        n1257 = call "IMAGE ANALYSIS.vi"("Enum"=POST_ANALYSIS_ENUM."SHOW UI", "error in"=w1402) -> ("error out"=w1400:errorcluster)  [unwired: 8 in, 1 out]
        n1258 = local write "Zoom Factore"(100.0 ("Zoom Factore")) -> ()
        n1259 = Strip Path(path=w1392) -> (name=w1395:string)  [unwired: 1 out]
        n1260 = Match Pattern(string=w1395, regular expression=w1393) -> (match substring=w1394:string)  [unwired: 1 in, 3 out]
        n1261 = Equal?(x=w1394, y=w1393) -> (x = y?=w1391:bool)
        n1262 = case shown="False" w1391 {
          frame False {
            n1263 = local write "Magnification :"("10x" ("Magnification :")) -> ()
          }
          frame True {
            n1264 = local write "Magnification :"("5x" ("Magnification :")) -> ()
          }
        }
      }
    }
    n1265 = case shown="True" w1086 {
      selector: w1086 -> [_ w1374]
      tunnel: w1078 -> [w1371 w1379]
      tunnel: [w1371 w1373] -> _
      frame False {
      }
      frame True {
        n1266 = Not(x=w1374) -> (.not. x?=w1372:bool)
        n1267 = local read "Zoom Factore"() -> (w1377:dbl)
        n1268 = local write "OUT"(w1372) -> ()
        n1269 = call "IMAGE ANALYSIS.vi"("Enum"=POST_ANALYSIS_ENUM."ZOOM OUT", "error in"=w1379) -> ("error out"=w1373:errorcluster)  [unwired: 8 in, 1 out]
        n1270 = Divide(x=w1377, y=1.2) -> (x/y=w1375:dbl)
        n1271 = local write "Zoom Factore"(w1375) -> ()
      }
    }
    n1272 = case shown="True" w1087 {
      selector: w1087 -> [_ w1383]
      tunnel: w1078 -> [w1380 w1388]
      tunnel: [w1380 w1381] -> _
      frame False {
      }
      frame True {
        n1273 = Not(x=w1383) -> (.not. x?=w1382:bool)
        n1274 = local read "Zoom Factore"() -> (w1386:dbl)
        n1275 = local write "In"(w1382) -> ()
        n1276 = call "IMAGE ANALYSIS.vi"("Enum"=POST_ANALYSIS_ENUM."ZOOM IN", "error in"=w1388) -> ("error out"=w1381:errorcluster)  [unwired: 8 in, 1 out]
        n1277 = Multiply(x=w1386, y=1.2) -> (x*y=w1384:dbl)
        n1278 = local write "Zoom Factore"(w1384) -> ()
      }
    }
    n1279 = case shown="True" w1083 {
      selector: w1083 -> [_ w1355]
      tunnel: w1078 -> [w1353 w1357]
      tunnel: [w1353 w1356] -> _
      frame False {
      }
      frame True {
        n1280 = Not(x=w1355) -> (.not. x?=w1354:bool)
        n1281 = local write "Clear ROI Tool"(w1354) -> ()
        n1282 = call "IMAGE ANALYSIS.vi"("Enum"=POST_ANALYSIS_ENUM."CLEAR ROI", "error in"=w1357) -> ("error out"=w1356:errorcluster)  [unwired: 8 in, 1 out]
      }
    }
    n1283 = case shown="True" w1085 {
      selector: w1085 -> [_ w1367]
      tunnel: w1078 -> [w1365 w1370]
      tunnel: [w1365 w1368] -> _
      frame False {
      }
      frame True {
        n1284 = Not(x=w1367) -> (.not. x?=w1366:bool)
        n1285 = local write "line tool"(w1366) -> ()
        n1286 = call "IMAGE ANALYSIS.vi"("Enum"=POST_ANALYSIS_ENUM."DRAW LINE", "error in"=w1370) -> ("error out"=w1368:errorcluster)  [unwired: 8 in, 1 out]
      }
    }
    n1287 = case shown="True" w1084 {
      selector: w1084 -> [_ w1361]
      tunnel: w1078 -> [w1359 w1363]
      tunnel: [w1359 w1362] -> _
      frame False {
      }
      frame True {
        n1288 = Not(x=w1361) -> (.not. x?=w1360:bool)
        n1289 = local write "Rectangle Tool"(w1360) -> ()
        n1290 = call "IMAGE ANALYSIS.vi"("Enum"=POST_ANALYSIS_ENUM."DRAW REC", "error in"=w1363) -> ("error out"=w1362:errorcluster)  [unwired: 8 in, 1 out]
      }
    }
    n1291 = local read "SCAR MEASURMENT"() -> (w1071:enum32{"Auto Scar", "Manual Scar"})
    n1292 = local read "Fit to Screen Tool"() -> (w1080:bool)
    n1293 = local read "Resize Tool"() -> (w1079:bool)
    n1294 = case shown="\"Manual Scar\", Default" w1071 {
      frame "Auto Scar" {
        n1295 = property on="Cap Live Image" class="Bool (strict)"("BoolText.Text"="Report" ("Boolean Text.Text")) -> ()  [unwired: 2 in, 2 out]
      }
      frame "Manual Scar", Default {
        n1296 = property on="Cap Live Image" class="Bool (strict)"("BoolText.Text"="Save Image" ("Boolean Text.Text")) -> ()  [unwired: 2 in, 2 out]
      }
    }
    n1297 = local read "ROI Color Tool"() -> (w1081:bool)
    n1298 = local read "Pan Tool"() -> (w1082:bool)
    n1299 = case shown="True" w1082 {
      selector: w1082 -> [_ w1349]
      tunnel: w1078 -> [w1347 w1351]
      tunnel: [w1347 w1350] -> _
      frame False {
      }
      frame True {
        n1300 = Not(x=w1349) -> (.not. x?=w1348:bool)
        n1301 = call "IMAGE ANALYSIS.vi"("Enum"=POST_ANALYSIS_ENUM."PAN", "error in"=w1351) -> ("error out"=w1350:errorcluster)  [unwired: 8 in, 1 out]
        n1302 = local write "Pan Tool"(w1348) -> ()
      }
    }
    n1303 = case shown="True" w1079 {
      selector: w1079 -> [_ w1333]
      tunnel: w1078 -> [w1328 w1330]
      tunnel: [w1328 w1329] -> _
      frame False {
      }
      frame True {
        n1304 = Not(x=w1333) -> (.not. x?=w1332:bool)
        n1305 = local write "Resize Tool"(w1332) -> ()
        n1306 = call "IMAGE ANALYSIS.vi"("Enum"=POST_ANALYSIS_ENUM."RESIZE MODE", "error in"=w1330) -> ("error out"=w1329:errorcluster)  [unwired: 8 in, 1 out]
      }
    }
    n1307 = case shown="True" w1080 {
      selector: w1080 -> [_ w1338]
      tunnel: [w1334 w1339] -> _
      tunnel: w1078 -> [w1334 w1337]
      frame False {
      }
      frame True {
        n1308 = Not(x=w1338) -> (.not. x?=w1336:bool)
        n1309 = local write "Zoom Factore"(100.0 ("Zoom Factore")) -> ()
        n1310 = local write "Fit to Screen Tool"(w1336) -> ()
        n1311 = call "IMAGE ANALYSIS.vi"("Enum"=POST_ANALYSIS_ENUM."FIT", "error in"=w1337) -> ("error out"=w1339:errorcluster)  [unwired: 8 in, 1 out]
      }
    }
    n1312 = case shown="True" w1081 {
      selector: w1081 -> [_ w1344]
      tunnel: [w1341 w1345] -> _
      tunnel: w1078 -> [w1341 w1342]
      frame False {
      }
      frame True {
        n1313 = Not(x=w1344) -> (.not. x?=w1343:bool)
        n1314 = local write "ROI Color Tool"(w1343) -> ()
        n1315 = call "IMAGE ANALYSIS.vi"("Enum"=POST_ANALYSIS_ENUM."SET ROI COLOR", "error in"=w1342) -> ("error out"=w1345:errorcluster)  [unwired: 8 in, 1 out]
      }
    }
    n1316 = local read "Quit"() -> (w1095:bool)
  }
  n1317 = while {
    stop <- w1440 stop-if-true
    n1318 = local read "Image Path"() -> (w1443:path)
    n1319 = local read "Print 3"() -> (w1446:bool)
    n1320 = Equal?(x=w1443, y=path "") -> (x = y?=w1442:bool)
    n1321 = Not(x=w1442) -> (.not. x?=w1441:bool)
    n1322 = property on="Print 3" class="Bool (strict)"("Visible"=w1441) -> ()  [unwired: 2 in, 2 out]
    n1323 = case shown="True" w1446 {
      frame False {
        n1324 = local write "Rd"(TRUE ("Boolean 7")) -> ()
      }
      frame True {
        n1325 = flat-sequence {
          tunnel: [w1486] -> w1454
          tunnel: [w1473] -> w1452
          tunnel: [w1483] -> w1448
          tunnel: w1454 -> [w1495]
          tunnel: [w1495] -> w1453
          tunnel: w1452 -> [w1494]
          tunnel: [w1494] -> w1451
          tunnel: [w1492] -> w1450
          tunnel: [w1491] -> w1449
          tunnel: w1448 -> [w1491]
          tunnel: w1453 -> [w1497]
          tunnel: w1451 -> [w1498]
          tunnel: w1450 -> [_]
          tunnel: w1449 -> [w1496]
          frame #0 {
            n1326 = case shown="True" "Rd" {
              frame False {
              }
              frame True {
                n1327 = while {
                  tunnel: "abcdefABCDEF" ("string 2") -> [w1465]
                  shift-right: [w1463] -> w1457
                  shift-left: "" -> [w1462]
                  i -> [w1472]
                  stop <- w1471 stop-if-true
                  n1328 = Random Number (0-1)() -> (number: 0 to 1=w1466:dbl)
                  n1329 = Multiply(x=w1466, y=62.0) -> (x*y=w1468:dbl)
                  n1330 = Decrement(x="Length 2") -> (x-1=w1461:i16)
                  n1331 = To Word Integer(number=w1468) -> (16bit integer=w1469:i16)
                  n1332 = String Subset(string=w1465, offset (0)=w1469, length (rest)=1 ("length (rest)")) -> (substring=w1464:string)
                  n1333 = Greater Or Equal?(x=w1472, y=w1461) -> (x >= y?=w1471:bool)
                  n1334 = Concatenate Strings(w1464, w1462) -> (w1463:string)
                }
                "String 10" <- w1457
                n1335 = local write "Rd"(FALSE ("Boolean 7")) -> ()
              }
            }
          }
          frame #1 {
            w1484 = "_resized.jpg" ("command line")
            (unwired) ".jpg -resize 320x240 " ("string")
            (unwired) "Choose an Image File" ("prompt")
            # "-resize 1798x425"
            n1336 = local read "Image Path"() -> (w1478:path)
            n1337 = Strip Path(path=w1478) -> (stripped path=w1473:path, name=w1474:string)
            n1338 = Match Pattern(string=w1474, regular expression=".jpg") -> (before substring=→"before substring 2":string, after substring=→"after substring":string)  [unwired: 1 in, 2 out]
            n1339 = Match Pattern(string=w1474, regular expression="\\") -> (before substring=w1480:string)  [unwired: 1 in, 3 out]
            n1340 = Match Pattern(string=w1480, regular expression=".jpg") -> (before substring=w1479:string)  [unwired: 1 in, 3 out]
            n1341 = Concatenate Strings("cmd /c convert " ("string"), w1479, ".jpg -resize 320x240  " ("command line"), w1479, w1484) -> (w1487:string)
            n1342 = call <vilib>:"System Exec.vi"("run minimized? (F)"=TRUE, "wait until completion? (T)"=TRUE, "working directory"=w1473, "command line"=w1487) -> ("error out"=w1486:errorcluster)  [unwired: 4 in, 3 out]
            "error out 2" <- w1486
            n1343 = Concatenate Strings(w1479, w1484) -> (w1483:string)
          }
          frame #2 {
            n1344 = Wait (ms)(milliseconds to wait=u32 2000 ("millisecond timer value")) -> (millisecond timer value=w1492:u32)
          }
          frame #3 {
            n1345 = case shown="No Error" w1497 {
              tunnel: w1498 -> [w1501 _]
              tunnel: w1496 -> [w1499 _]
              frame No Error {
                (unwired) ".jpg" ("string")
                n1346 = Path To String(path=w1501) -> (string=w1505:string)
                n1347 = Concatenate Strings(w1505, "\\" ("string"), w1499) -> (w1504:string)
                n1348 = String To Path(string=w1504) -> (path=w1503:path)
                n1349 = call <vilib>:"Read JPEG File.vi"("path to JPEG file"=w1503) -> ("image data"=w1507:T2)  [unwired: 8 in, 2 out]